vi "HFRR ADV v039 new software.vi"() -> ()   [LabVIEW 2025] (continued)
                n2173 = Number To Fractional String(number=w2771, width (-)=i16 10 ("precision (6)"), precision (6)=i16 5) -> (F-format string=w2865:string)  [unwired: 1 in]
                n2174 = Number To Fractional String(number=w2771, width (-)=i16 10 ("precision (6)"), precision (6)=i16 5) -> (F-format string=w2866:string)  [unwired: 1 in]
                n2175 = Concatenate Strings("[CHH]" ("string"), w2792, "-Humidity Dry" ("string"), "\r") -> (w2786:string)
                n2176 = Concatenate Strings("[CHG]" ("string"), w2797, "-Humidity Wet" ("string"), "\r") -> (w2787:string)
                n2177 = Concatenate Strings("[CHD]" ("string"), w2808, "-Power +" ("string"), "\r") -> (w2790:string)
                n2178 = Concatenate Strings("[CHC]" ("string"), w2814, "-Language Selection" ("string"), "\r") -> (w2811:string)
                n2179 = Concatenate Strings("[CHA]" ("string"), w2825, "- Stroke Gain" ("string"), "\r") -> (w2819:string)
                n2180 = Concatenate Strings("[CHF]" ("string"), w2800, "-Heater" ("string"), "\r") -> (w2788:string)
                n2181 = Concatenate Strings("[CHE]" ("string"), w2805, "-Power_" ("string"), "\r") -> (w2789:string)
                n2182 = Concatenate Strings("[CH8]" ("string"), w2826, "- Displacement Gain" ("string"), "\r") -> (w2829:string)
                n2183 = Concatenate Strings("[CH7]" ("string"), w2833, "- file path" ("string"), "\r") -> (w2836:string)
                n2184 = Concatenate Strings("[CH6]" ("string"), w2773, "- Visa Due" ("string"), "\r") -> (w2837:string)
                n2185 = Concatenate Strings("[CH5]" ("string"), w2774, "- Visa Uno" ("string"), "\r") -> (w2842:string)
                n2186 = Concatenate Strings("[CH4]" ("string"), w2853, " - AIR TEMP" ("string"), "\r") -> (w2849:string)
                n2187 = Concatenate Strings("[CH3]" ("string"), w2859, " - Humidity" ("string"), "\r") -> (w2856:string)
                n2188 = Concatenate Strings("[CH2]" ("string"), w2865, " - TEMPERATURE" ("string"), "\r") -> (w2863:string)
                n2189 = Concatenate Strings("[CH1]" ("string"), w2866, " - FF" ("string"), "\r") -> (w2864:string)
                n2190 = Concatenate Strings(w2864, w2863, w2856, w2849, w2842, w2837, w2836, w2829, w2819, w2811, w2790, w2789, w2788, w2787, w2786) -> (w2775:string)
                "gain" <- w2775
              }
              frame #1 {
                w2877 = 0.0 ("number")
                n2191 = local read "Camera Port :"() -> (w2880:string)
                n2192 = local read "C3 :"() -> (w2888:refnum<visa-resource-name>)
                n2193 = local read "Com Port 3"() -> (w2889:refnum<visa-resource-name>)
                n2194 = Concatenate Strings("[CH8]" ("string"), w2880, "- Visa Camera" ("string"), "\r") -> (w2879:string)
                n2195 = Concatenate Strings("[CH7]" ("string"), w2888, "- Visa Humidity" ("string"), "\r") -> (w2884:string)
                n2196 = Number To Fractional String(number=w2877, width (-)=i16 10 ("precision (6)"), precision (6)=i16 5) -> (F-format string=w2904:string)  [unwired: 1 in]
                n2197 = Concatenate Strings("[CHL]" ("string"), w2889, "- Visa humid" ("string"), "\r") -> (w2892:string)
                n2198 = Number To Fractional String(number=w2877, width (-)=i16 10 ("precision (6)"), precision (6)=i16 5) -> (F-format string=w2911:string)  [unwired: 1 in]
                n2199 = Concatenate Strings("[SNO]" ("string"), "" ("string"), "-" ("string"), "\r") -> (w2897:string)
                n2200 = Concatenate Strings("[CHK]" ("string"), w2904, "-TEMP INTERCEPT" ("string"), "\r") -> (w2900:string)
                n2201 = Concatenate Strings("[CHJ]" ("string"), w2911, "-AIR TEMP INTERCEPT" ("string"), "\r") -> (w2901:string)
                n2202 = String To Path(string="C:\\LAB-IQ\\calibrate WO 2465.dcf") -> (path=w2890:path)
                n2203 = Concatenate Strings(w2916, w2901, w2900, w2897, w2892, w2884, w2879) -> (w2915:string)
                n2204 = call <vilib>:"Write Characters To File.vi"("append to file? (new file:F)"=FALSE, "character string"=w2915, "file path (dialog if empty)"=w2890) -> ()  [unwired: 2 in, 1 out]
              }
              frame #2 {
                n2205 = local write "Lan flag"(0.0 ("Lan flag")) -> ()
                n2206 = local write "conststatus"(0.0 ("rpm value : 2")) -> ()
                n2207 = local write "SAVE"(FALSE ("OK Button 14")) -> ()
              }
            }
          }
        }
        n2208 = property on="Language Selection" class="Enum (strict)"("Visible"=w2712) -> ()  [unwired: 2 in, 2 out]
        n2209 = property on="SPEED OUT:" class="DigNum (strict)"("Disabled"=w2713) -> ()  [unwired: 2 in, 2 out]
      }
    }
    n2210 = case shown="False" w2239 {
      frame False {
        n2211 = local read "stopT"() -> (w2927:bool)
        n2212 = case shown="True" w2927 {
          frame False {
          }
          frame True {
            n2213 = local write "stopT"(FALSE) -> ()
          }
        }
      }
      frame True {
        "stopT" <- TRUE
      }
    }
    n2214 = case shown="True" w2229 {
      frame False {
        n2215 = property on="Password 2" class="Str"("Visible"=FALSE) -> ()  [unwired: 2 in, 2 out]
        n2216 = local write "Password 2"("" ("Password")) -> ()
      }
      frame True {
        n2217 = property on="Password 2" class="Str"("Visible"=TRUE) -> ()  [unwired: 2 in, 2 out]
        n2218 = Equal?(x="Password 2", y="HFRR1234") -> (x = y?=w2252:bool)
        n2219 = case shown="True" w2252 {
          tunnel: "Password 2" -> [w2255 _]
          frame False {
            n2220 = String Length(string=w2255) -> (length=w2256:i32)
            n2221 = Greater Than 0?(x=w2256) -> (x > 0?=w2254:bool)
            n2222 = case shown="False" w2254 {
              frame False {
                n2223 = property on="Password 2" class="Str"("Caption.Text"="Password (Advance Setting)") -> ()  [unwired: 2 in, 2 out]
              }
              frame True {
                n2224 = property on="Password 2" class="Str"("Caption.Text"="Incorrect Password!") -> ()  [unwired: 2 in, 2 out]
              }
            }
          }
          frame True {
            n2225 = local write "EDIT 2"(FALSE ("EDIT 2")) -> ()
            n2226 = local write "Password 2"("" ("Password")) -> ()
            n2227 = local write "Main Tab"(T2."Advance" ("Main Tab")) -> ()
            n2228 = local write "Main Dashboard Buttons"(T1."Advance" ("Main Dashboard Buttons")) -> ()
          }
        }
      }
    }
    n2229 = case shown="\"Acquire\", Default" w2235 {
      frame "Acquire", Default {
        # "Elapsed time\ncof\nstroke\nAir temp\nTemp\nHumidity"
        n2230 = local read "RUN"() -> (w2934:bool)
        n2231 = stacked-sequence {
          frame #0 {
            n2232 = case shown="True" "RST FF" {
              frame False {
              }
              frame True {
                w3011 = 0.0 ("X Scale.Range:Maximum")
                n2233 = property on="Frictional Force ( N )" class="WFChart (strict)"("XScale.Maximum"=600.0 ("X Scale.Range:Maximum"), "XScale.Minimum"=w3011, "YScale.Maximum"=10.0 ("Y Scale.Range:Maximum"), "YScale.Minimum"=w3011) -> ()  [unwired: 2 in, 2 out]
              }
            }
          }
          frame #1 {
            n2234 = case shown="True" "RST TEMP" {
              frame False {
              }
              frame True {
                n2235 = property on="Temperature ( Deg C )" class="WFChart (strict)"("XScale.Minimum"=0.0 ("X Scale.Range:Minimum"), "XScale.Maximum"=600.0 ("X Scale.Range:Maximum"), "YScale.Minimum"=0.0 ("Y Scale.Range:Minimum"), "YScale.Maximum"=100.0 ("Y Scale.Range:Maximum")) -> ()  [unwired: 2 in, 2 out]
              }
            }
          }
          frame #2 {
            n2236 = case shown="True" "RSTCOF" {
              frame False {
              }
              frame True {
                n2237 = property on="Coefficient of Friction" class="WFChart (strict)"("XScale.Minimum"=0.0 ("X Scale.Range:Minimum"), "XScale.Maximum"=600.0 ("X Scale.Range:Maximum"), "YScale.Maximum"=1.0 ("X Scale.Range:Minimum"), "YScale.Minimum"=0.0 ("X Scale.Range:Minimum")) -> ()  [unwired: 2 in, 2 out]
              }
            }
          }
          frame #3 {
            n2238 = case shown="True" "RSTCOF 2" {
              frame False {
              }
              frame True {
                (unwired) 100.0 ("Y Scale.Range:Maximum")
                (unwired) 0.0 ("Y Scale.Range:Minimum")
                (unwired) 600.0 ("X Scale.Range:Maximum")
                (unwired) 0.0 ("X Scale.Range:Minimum")
              }
            }
          }
          frame #4 {
            n2239 = case shown="True" "RSTCOF 3" {
              frame False {
              }
              frame True {
                n2240 = property on="Electrical Contact Resistance ( % )" class="WFChart (strict)"("XScale.Minimum"=0.0 ("X Scale.Range:Minimum"), "XScale.Maximum"=600.0 ("X Scale.Range:Maximum"), "YScale.Minimum"=0.0 ("Y Scale.Range:Minimum"), "YScale.Maximum"=100.0 ("Y Scale.Range:Maximum")) -> ()  [unwired: 2 in, 2 out]
              }
            }
          }
        }
        n2241 = case shown="False" w2934 {
          frame False {
          }
          frame True {
          }
        }
        n2242 = disable-structure shown="Disabled" {
          frame Disabled {
            n2243 = local read "RUN"() -> (w2941:bool)
            n2244 = local read "Flag"() -> (w2944:dbl)
            n2245 = Not(x=w2941) -> (.not. x?=w2940:bool)
            n2246 = Equal?(x=w2944, y=10.0) -> (x = y?=w2942:bool)
            n2247 = And(x=w2942, y=w2940) -> (x .and. y?=w2939:bool)
            n2248 = case shown="True" w2939 {
              frame False {
              }
              frame True {
                w2945 = FALSE ("Heater Button")
                n2249 = local write "Humidity"(w2945) -> ()
                n2250 = local write "Heater Button"(w2945) -> ()
              }
            }
          }
          frame Enabled {
          }
        }
        n2251 = local read "RUN"() -> (w2938:bool)
        n2252 = case shown="False" w2938 {
          tunnel: [FALSE ("TEST RUNNING") TRUE ("TEST RUNNING")] -> w2937
          frame False {
            w3030 = 0.0 ("Flag")
            n2253 = local write "Elapsed time"(0.0 ("elapsedtime")) -> ()
            n2254 = local write "Time Remaining"(w3030) -> ()
            n2255 = local write "Flag"(w3030) -> ()
            n2256 = local write "Remaining Time"(w3030) -> ()
          }
          frame True {
            n2257 = local write "Flag"(10.0 ("Flag")) -> ()
          }
        }
        n2258 = local read "AIR TEMP"() -> (w2932:dbl)
        n2259 = Greater Or Equal?(x=w2932, y=15.0) -> (x >= y?=w2933:bool)
        "powstat" <- w2933
        n2260 = case shown="True" "Save & Continue" {
          frame False {
          }
          frame True {
            n2261 = local read "USER ID"() -> (w3339:string)
            n2262 = local read "FILE"() -> (w3347:string)
            n2263 = String Length(string=w3339) -> (length=w3342:i32)
            n2264 = String Length(string=w3347) -> (length=w3345:i32)
            n2265 = Greater?(x=w3342, y=0) -> (0:w3341:bool)
            n2266 = Greater?(x=w3345, y=0) -> (0:w3344:bool)
            n2267 = And(x=w3344, y=w3341) -> (x .and. y?=w3340:bool)
            n2268 = case shown="True" w3340 {
              frame False {
                n2269 = stacked-sequence {
                  frame #0 {
                    n2270 = One Button Dialog(message="Please Enter a File Name and Operator ID to save data !", button name ("OK")="Ok") -> ()  [unwired: 1 out]
                  }
                  frame #1 {
                    n2271 = local write "Save & Continue"(FALSE ("OK Button")) -> ()
                  }
                }
                n2272 = local write "Save & Continue"(FALSE ("OK Button")) -> ()
              }
              frame True {
                n2273 = stacked-sequence {
                  frame #0 {
                    n2274 = local read "FILE"() -> (w3353:string)
                    n2275 = call "file check.vi"("file name in"=w3353) -> ("file name out"=w3352:string)  [unwired: 9 in, 1 out]
                    n2276 = call <vilib>:"Application Directory.vi"() -> ("Application Directory"=w3363:path)
                    n2277 = Build Path(base path=w3363, name or relative path="data") -> (appended path=w3362:path)
                    n2278 = call <vilib>:"Trim Whitespace.vi"("string"=w3352) -> ("trimmed string"=w3360:string)  [unwired: 1 in]
                    n2279 = call <vilib>:"Trim Whitespace.vi"("string"=w3352) -> ("trimmed string"=w3361:string)  [unwired: 1 in]
                    n2280 = List Folder(path=w3362) -> (folder names=w3358:string[])  [unwired: 3 in, 3 out]
                    n2281 = Match Pattern(string=w3360, regular expression="_(") -> (before substring=w3357:string)  [unwired: 1 in, 3 out]
                    n2282 = Equal?(x=w3358, y=w3357) -> (x = y?=w3366:bool[])
                    n2283 = for {
                      tunnel: w3358 -> [w3372] mode=indexing
                      tunnel: w3357 -> [w3370]
                      shift-right: [w3368] -> w3355
                      shift-left: bool[] [] -> [w3369]
                      n2284 = Match Pattern(string=w3372, regular expression="_(") -> (before substring=w3371:string)  [unwired: 1 in, 3 out]
                      n2285 = Equal?(x=w3371, y=w3370) -> (x = y?=w3367:bool)
                      n2286 = case shown="True" w3367 {
                        tunnel: w3367 -> [_ w3375]
                        tunnel: w3369 -> [w3374 w3377]
                        tunnel: [w3374 w3376] -> w3368
                        frame False {
                        }
                        frame True {
                          n2287 = Insert Into Array(array=w3377, new element=w3375) -> (w3376:bool[])  [unwired: 1 in]
                        }
                      }
                    }
                    n2288 = Or Array Elements(Boolean array=w3366) -> (logical OR=w3365:bool)
                    n2289 = Array Size(array=w3355) -> (size(s)=w3354:i32)
                    n2290 = case shown="True" w3365 {
                      tunnel: w3361 -> [_ w3385]
                      tunnel: w3354 -> [_ w3378]
                      frame False {
                      }
                      frame True {
                        n2291 = Number To Decimal String(number=w3378) -> (decimal integer string=w3381:string)  [unwired: 1 in]
                        n2292 = Search/Split String(string=w3385, search string/char (-)="_(" ("regular expression")) -> (substring before match=w3383:string)  [unwired: 1 in, 2 out]
                        n2293 = Concatenate Strings(w3383, "_(" ("regular expression"), w3381, ")" ("regular expression")) -> (w3379:string)
                        n2294 = local write "FILE"(w3379) -> ()
                      }
                    }
                  }
                  frame #1 {
                    w3388 = 0.0
                    w3401 = cluster{"y":dbl, dbl, "y":dbl}[] [] ("History Data")
                    w3402 = FALSE ("Heater Button")
                    (unwired) ")!" ("string")
                    (unwired) ")" ("string")
                    w3400 = dbl[] [] ("History Data")
                    w3406 = "\r"
                    # "C:\\WinDucom\\Data\\"
                    # "C:\\LAB-IQ-NXT\\data"
                    n2295 = local write "Humidity ( %RH )"(w3388) -> ()
                    n2296 = local write "Frequency ( Hz )"(w3388) -> ()
                    n2297 = local write "Stroke 3"(w3388) -> ()
                    n2298 = local write "Set Temp 2"(65.0 ("Set Temp 2")) -> ()
                    n2299 = local write "speedop"(0.0 ("PIDclk 2")) -> ()
                    n2300 = local write "AIR TEMP"(w3388) -> ()
                    n2301 = local write "Stroke 4"(w3388) -> ()
                    n2302 = local write "clk"(0.0 ("clk")) -> ()
                    n2303 = local write "COF 2"(w3388) -> ()
                    n2304 = local write "TEMP"(w3388) -> ()
                    n2305 = local write "ecr 3"(w3388) -> ()
                    n2306 = local write "FF 2"(w3388) -> ()
                    n2307 = local write "FF 3"(w3388) -> ()
                    n2308 = property on="Temperature ( Deg C )" class="WFChart (strict)"("History Data"=w3400) -> ()  [unwired: 2 in, 2 out]
                    n2309 = property on="Electrical Contact Resistance ( % )" class="WFChart (strict)"("History Data"=w3400) -> ()  [unwired: 2 in, 2 out]
                    n2310 = property on="Frictional Force ( N )" class="WFChart (strict)"("History Data"=w3400) -> ()  [unwired: 2 in, 2 out]
                    n2311 = property on="Coefficient of Friction" class="WFChart (strict)"("History Data"=w3400) -> ()  [unwired: 2 in, 2 out]
                    n2312 = property on="Humidity ( %RH ) 2" class="WFChart (strict)"("History Data"=w3400) -> ()  [unwired: 2 in, 2 out]
                    n2313 = property on="Temperature ( Deg C )" class="WFChart (strict)"("History Data"=w3400) -> ()  [unwired: 2 in, 2 out]
                    n2314 = property on="Electrical Contact Resistance ( % )" class="WFChart (strict)"("History Data"=w3400) -> ()  [unwired: 2 in, 2 out]
                    n2315 = property on="Frictional Force ( N )" class="WFChart (strict)"("History Data"=w3400) -> ()  [unwired: 2 in, 2 out]
                    n2316 = property on="Coefficient of Friction" class="WFChart (strict)"("History Data"=w3400) -> ()  [unwired: 2 in, 2 out]
                    n2317 = property on="Electrical Contact Resistance ( % )" class="WFChart (strict)"("History Data"=w3400) -> ()  [unwired: 2 in, 2 out]
                    n2318 = property on="Frictional Force ( N )" class="WFChart (strict)"("History Data"=w3400) -> ()  [unwired: 2 in, 2 out]
                    n2319 = property on="Coefficient of Friction" class="WFChart (strict)"("History Data"=w3400) -> ()  [unwired: 2 in, 2 out]
                    n2320 = property on="Stroke ( mm )" class="WFChart (strict)"("History Data"=w3401) -> ()  [unwired: 2 in, 2 out]
                    n2321 = property on="Stroke ( mm )" class="WFChart (strict)"("History Data"=w3401) -> ()  [unwired: 2 in, 2 out]
                    n2322 = local write "Humidity"(w3402) -> ()
                    n2323 = local write "Heater Button"(w3402) -> ()
                    n2324 = local read "FILE"() -> (w3396:string)
                    n2325 = disable-structure shown="Enabled" {
                      disable-tunnel: [w3440 _] -> w3387
                      frame Enabled {
                        n2326 = local read "NORMAL LOAD"() -> (w3440:dbl)
                      }
                      frame Disabled {
                      }
                    }
                    n2327 = call "file check.vi"("file name in"=w3396) -> ("error out"=w3399:errorcluster, "file name out"=w3393:string)  [unwired: 9 in]
                    n2328 = call "FILE PATH CREATION.vi"("error in"=w3399, "FILE NAME :"=w3393) -> ("FILE OUT"=w3392:path)  [unwired: 8 in, 1 out]
                    n2329 = Concatenate Strings(w3393, ".dgf" ("Substring")) -> (w3398:string)
                    n2330 = Concatenate Strings(w3393, ".duf" ("Substring")) -> (w3394:string)
                    n2331 = Multiply(x=w3387, y=1.0) -> (x*y=w3419:dbl)
                    n2332 = Build Path(base path=w3392, name or relative path=w3398) -> (appended path=w3391:path)
                    n2333 = Build Path(base path=w3392, name or relative path=w3394) -> (appended path=w3390:path)
                    n2334 = Number To Fractional String(number=w3419, width (-)=i16 5, precision (6)=i16 2) -> (F-format string=w3427:string)  [unwired: 1 in]
                    n2335 = local read "tested by"() -> (w3386:string)
                    n2336 = local read "Fuel Discription :"() -> (w3415:string)
                    n2337 = local read "Batch Ref Num :"() -> (w3404:string)
                    n2338 = Get Date/Time String(date format (0)=enum16{"short", "long", "abbreviated"}."short") -> (date string=w3438:string, time string=w3435:string)  [unwired: 2 in]
                    n2339 = local read "Remarks :"() -> (w3414:string)
                    n2340 = Concatenate Strings("Load :- " ("Substring"), w3427, " grams ," ("Substring")) -> (w3426:string)
                    n2341 = local read "String 41"() -> (w3407:string)
                    n2342 = Concatenate Strings(w3404) -> (w3403:string)
                    n2343 = Concatenate Strings(w3386) -> (w3410:string)
                    n2344 = Concatenate Strings(w3415) -> (w3416:string)
                    n2345 = Concatenate Strings("(" ("Substring"), w3438, ")" ("Substring"), w3435) -> (w3409:string)
                    "concatenated string" <- w3409
                    n2346 = Concatenate Strings(w3414, "," ("string")) -> (w3413:string)
                    n2347 = Concatenate Strings("  TIME;      COF;       STROKE;     AIR TEMP;  TEMP;  HUMIDITY;  ECR; PID-OUT; FREQUENCY" ("Substring"), "\r") -> (w3422:string)
                    n2348 = Concatenate Strings(w3407, w3406, "Fuel Discription :-" ("Substring"), w3416, w3406, w3426, w3406, "Batch Ref Num :-" ("Substring"), w3403, w3406, " Remarks :- " ("Substring"), w3413, w3406, " Date :- " ("Substring"), w3409, w3406, "Tested By :-" ("Substring"), w3410) -> (w3420:string)
                    "REMARKS" <- w3420
                    n2349 = call <vilib>:"Write Characters To File.vi"("append to file? (new file:F)"=FALSE, "character string"=w3420, "file path (dialog if empty)"=w3390) -> ()  [unwired: 2 in, 1 out]
                    n2350 = call <vilib>:"Write Characters To File.vi"("append to file? (new file:F)"=FALSE, "character string"=w3422, "file path (dialog if empty)"=w3391) -> ()  [unwired: 2 in, 1 out]
                  }
                  frame #2 {
                    n2351 = local write "Cycles elapsed"(0 ("Cycles elapsed")) -> ()
                    n2352 = local write "cyclecount"(0 ("cyclecount")) -> ()
                    n2353 = local write "autostrtflg"(TRUE ("autostrtflg")) -> ()
                    n2354 = local write "Save"(FALSE ("Save")) -> ()
                    n2355 = local write "Save & Continue"(FALSE ("OK")) -> ()
                    n2356 = Get Date/Time In Seconds() -> (seconds since 1Jan1904=w3445:timestamp)
                    n2357 = To Double Precision Float(number=w3445) -> (double precision float=w3444:dbl)
                    n2358 = local write "acq timer"(w3444) -> ()
                    n2359 = One Button Dialog(message="Please ensure sample is mounted properly and machine is ready in all aspects for testing !", button name ("OK")="Ok") -> ()  [unwired: 1 out]
                  }
                  frame #3 {
                    n2360 = stacked-sequence {
                      frame #0 {
                        n2361 = local write "Main Dashboard Buttons"(T1."Dashboard" ("Main Dashboard Buttons")) -> ()
                        n2362 = local write "Main Tab"(T2."Acquire" ("Main Tab")) -> ()
                      }
                      frame #1 {
                        n2363 = local write "EVENT LOG"("" ("EVENT LOG")) -> ()
                      }
                      frame #2 {
                        n2364 = Wait (ms)(milliseconds to wait=u32 50) -> ()  [unwired: 1 out]
                      }
                      frame #3 {
                        n2365 = disable-structure shown="Disabled" {
                          frame Disabled {
                            n2366 = local read "EVENT LOG"() -> (w3457:string)
                            n2367 = call "Event Log.vi"("Content"="Test Details", "EVENT LOG"=w3457) -> ("EVENT LOG"=w3456:string)  [unwired: 8 in, 1 out]
                            n2368 = local write "EVENT LOG"(w3456) -> ()
                          }
                          frame Enabled {
                          }
                        }
                      }
                      frame #4 {
                        n2369 = Wait (ms)(milliseconds to wait=u32 50) -> ()  [unwired: 1 out]
                      }
                      frame #5 {
                        n2370 = local read "FILE"() -> (w3459:string)
                        n2371 = Concatenate Strings("File Name :" ("Content"), w3459) -> (w3460:string)
                        n2372 = local read "EVENT LOG"() -> (w3463:string)
                        n2373 = call "Event Log.vi"("Content"=w3460, "EVENT LOG"=w3463) -> ("EVENT LOG"=w3462:string)  [unwired: 8 in, 1 out]
                        n2374 = local write "EVENT LOG"(w3462) -> ()
                      }
                      frame #6 {
                        n2375 = Wait (ms)(milliseconds to wait=u32 50) -> ()  [unwired: 1 out]
                      }
                      frame #7 {
                        n2376 = local read "Batch Ref Num :"() -> (w3465:string)
                        n2377 = Concatenate Strings("Batch Ref No :" ("Content"), w3465) -> (w3466:string)
                        n2378 = local read "EVENT LOG"() -> (w3469:string)
                        n2379 = call "Event Log.vi"("Content"=w3466, "EVENT LOG"=w3469) -> ("EVENT LOG"=w3468:string)  [unwired: 8 in, 1 out]
                        n2380 = local write "EVENT LOG"(w3468) -> ()
                      }
                      frame #8 {
                        n2381 = Wait (ms)(milliseconds to wait=u32 50) -> ()  [unwired: 1 out]
                      }
                      frame #9 {
                        n2382 = local read "tested by"() -> (w3471:string)
                        n2383 = Concatenate Strings("Tested By :" ("Content"), w3471) -> (w3472:string)
                        n2384 = local read "EVENT LOG"() -> (w3475:string)
                        n2385 = call "Event Log.vi"("Content"=w3472, "EVENT LOG"=w3475) -> ("EVENT LOG"=w3474:string)  [unwired: 8 in, 1 out]
                        n2386 = local write "EVENT LOG"(w3474) -> ()
                      }
                      frame #10 {
                        n2387 = Wait (ms)(milliseconds to wait=u32 50) -> ()  [unwired: 1 out]
                      }
                      frame #11 {
                        n2388 = local read "TEST STANDARD"() -> (w3478:T3)
                        n2389 = case shown="\"ASTM D6079\", Default" w3478 {
                          tunnel: ["ASTM D6079" "ISO 12156" "CEC F-096-A-06" "Custom"] -> w3477
                          frame "ASTM D6079", Default {
                          }
                          frame "ISO 12156" {
                          }
                          frame "CEC F-096-A-06" {
                          }
                          frame "Custom" {
                          }
                        }
                        n2390 = Concatenate Strings("Test Standard :" ("Content"), w3477) -> (w3479:string)
                        n2391 = local read "EVENT LOG"() -> (w3482:string)
                        n2392 = call "Event Log.vi"("Content"=w3479, "EVENT LOG"=w3482) -> ("EVENT LOG"=w3481:string)  [unwired: 8 in, 1 out]
                        n2393 = local write "EVENT LOG"(w3481) -> ()
                      }
                      frame #12 {
                        n2394 = Wait (ms)(milliseconds to wait=u32 50) -> ()  [unwired: 1 out]
                      }
                      frame #13 {
                        n2395 = local read "Fuel Discription :"() -> (w3488:string)
                        n2396 = Concatenate Strings("Fuel Description :" ("Content"), w3488) -> (w3489:string)
                        n2397 = local read "EVENT LOG"() -> (w3492:string)
                        n2398 = call "Event Log.vi"("Content"=w3489, "EVENT LOG"=w3492) -> ("EVENT LOG"=w3491:string)  [unwired: 8 in, 1 out]
                        n2399 = local write "EVENT LOG"(w3491) -> ()
                      }
                      frame #14 {
                        n2400 = Wait (ms)(milliseconds to wait=u32 50) -> ()  [unwired: 1 out]
                      }
                      frame #15 {
                        n2401 = local read "Remarks :"() -> (w3494:string)
                        n2402 = Concatenate Strings("Remarks :" ("Content"), w3494) -> (w3495:string)
                        n2403 = local read "EVENT LOG"() -> (w3498:string)
                        n2404 = call "Event Log.vi"("Content"=w3495, "EVENT LOG"=w3498) -> ("EVENT LOG"=w3497:string)  [unwired: 8 in, 1 out]
                        n2405 = local write "EVENT LOG"(w3497) -> ()
                      }
                      frame #16 {
                        n2406 = Wait (ms)(milliseconds to wait=u32 50) -> ()  [unwired: 1 out]
                      }
                      frame #17 {
                        n2407 = local read "USER ID"() -> (w3500:string)
                        n2408 = Concatenate Strings("Operator ID :" ("Content"), w3500) -> (w3502:string)
                        n2409 = local read "EVENT LOG"() -> (w3504:string)
                        n2410 = call "Event Log.vi"("Content"=w3502, "EVENT LOG"=w3504) -> ("EVENT LOG"=w3503:string)  [unwired: 8 in, 1 out]
                        n2411 = local write "EVENT LOG"(w3503) -> ()
                      }
                      frame #18 {
                        n2412 = Wait (ms)(milliseconds to wait=u32 50) -> ()  [unwired: 1 out]
                      }
                      frame #19 {
                        n2413 = disable-structure shown="Disabled" {
                          frame Disabled {
                            n2414 = local read "EVENT LOG"() -> (w3508:string)
                            n2415 = call "Event Log.vi"("Content"="Test Parameter", "EVENT LOG"=w3508) -> ("EVENT LOG"=w3507:string)  [unwired: 8 in, 1 out]
                            n2416 = local write "EVENT LOG"(w3507) -> ()
                          }
                          frame Enabled {
                          }
                        }
                      }
                      frame #20 {
                        n2417 = Wait (ms)(milliseconds to wait=u32 50) -> ()  [unwired: 1 out]
                      }
                      frame #21 {
                        n2418 = local read "Set Hz"() -> (w3512:dbl)
                        n2419 = Number To Fractional String(number=w3512, precision (6)=i16 2) -> (F-format string=w3511:string)  [unwired: 2 in]
                        n2420 = Concatenate Strings("Set Frequency [Hz] :" ("Content"), w3511) -> (w3514:string)
                        n2421 = local read "EVENT LOG"() -> (w3516:string)
                        n2422 = call "Event Log.vi"("Content"=w3514, "EVENT LOG"=w3516) -> ("EVENT LOG"=w3515:string)  [unwired: 8 in, 1 out]
                        n2423 = local write "EVENT LOG"(w3515) -> ()
                      }
                      frame #22 {
                        n2424 = Wait (ms)(milliseconds to wait=u32 50) -> ()  [unwired: 1 out]
                      }
                      frame #23 {
                        n2425 = local read "NORMAL LOAD"() -> (w3519:dbl)
                        n2426 = Number To Fractional String(number=w3519, precision (6)=i16 2) -> (F-format string=w3520:string)  [unwired: 2 in]
                        n2427 = Concatenate Strings("Applied Load [grams] :" ("Content"), w3520) -> (w3522:string)
                        n2428 = local read "EVENT LOG"() -> (w3524:string)
                        n2429 = call "Event Log.vi"("Content"=w3522, "EVENT LOG"=w3524) -> ("EVENT LOG"=w3523:string)  [unwired: 8 in, 1 out]
                        n2430 = local write "EVENT LOG"(w3523) -> ()
                      }
                      frame #24 {
                        n2431 = Wait (ms)(milliseconds to wait=u32 50) -> ()  [unwired: 1 out]
                      }
                      frame #25 {
                        n2432 = local read "Set Strk"() -> (w3527:dbl)
                        n2433 = Number To Fractional String(number=w3527, precision (6)=i16 2) -> (F-format string=w3528:string)  [unwired: 2 in]
                        n2434 = Concatenate Strings("Set Stroke [mm] :" ("Content"), w3528) -> (w3530:string)
                        n2435 = local read "EVENT LOG"() -> (w3532:string)
                        n2436 = call "Event Log.vi"("Content"=w3530, "EVENT LOG"=w3532) -> ("EVENT LOG"=w3531:string)  [unwired: 8 in, 1 out]
                        n2437 = local write "EVENT LOG"(w3531) -> ()
                      }
                      frame #26 {
                        n2438 = Wait (ms)(milliseconds to wait=u32 50) -> ()  [unwired: 1 out]
                      }
                      frame #27 {
                        n2439 = local read "Set Temp"() -> (w3535:dbl)
                        n2440 = Number To Fractional String(number=w3535, precision (6)=i16 2) -> (F-format string=w3536:string)  [unwired: 2 in]
                        n2441 = Concatenate Strings("Set Temperature [deg C] :" ("Content"), w3536) -> (w3538:string)
                        n2442 = local read "EVENT LOG"() -> (w3540:string)
                        n2443 = call "Event Log.vi"("Content"=w3538, "EVENT LOG"=w3540) -> ("EVENT LOG"=w3539:string)  [unwired: 8 in, 1 out]
                        n2444 = local write "EVENT LOG"(w3539) -> ()
                      }
                      frame #28 {
                        n2445 = Wait (ms)(milliseconds to wait=u32 50) -> ()  [unwired: 1 out]
                      }
                      frame #29 {
                        n2446 = local read "Set Rh"() -> (w3543:dbl)
                        n2447 = Number To Fractional String(number=w3543, precision (6)=i16 2) -> (F-format string=w3544:string)  [unwired: 2 in]
                        n2448 = Concatenate Strings("Set Humidity [%RH] :" ("Content"), w3544) -> (w3546:string)
                        n2449 = local read "EVENT LOG"() -> (w3548:string)
                        n2450 = call "Event Log.vi"("Content"=w3546, "EVENT LOG"=w3548) -> ("EVENT LOG"=w3547:string)  [unwired: 8 in, 1 out]
                        n2451 = local write "EVENT LOG"(w3547) -> ()
                      }
                      frame #30 {
                        n2452 = Wait (ms)(milliseconds to wait=u32 50) -> ()  [unwired: 1 out]
                      }
                      frame #31 {
                        n2453 = local read "test time"() -> (w3551:dbl)
                        n2454 = Number To Fractional String(number=w3551, precision (6)=i16 1) -> (F-format string=w3552:string)  [unwired: 2 in]
                        n2455 = Concatenate Strings("Test Duration [mins] :" ("Content"), w3552) -> (w3554:string)
                        n2456 = local read "EVENT LOG"() -> (w3556:string)
                        n2457 = call "Event Log.vi"("Content"=w3554, "EVENT LOG"=w3556) -> ("EVENT LOG"=w3555:string)  [unwired: 8 in, 1 out]
                        n2458 = local write "EVENT LOG"(w3555) -> ()
                      }
                      frame #32 {
                        w3557 = dbl[] [] ("History Data")
                        w3558 = cluster{"y":dbl, dbl, "y":dbl}[] [] ("History Data")
                        w3559 = FALSE ("Visible")
                        n2459 = property on="Stroke ( mm )" class="WFChart (strict)"("History Data"=w3558) -> ()  [unwired: 2 in, 2 out]
                        n2460 = property on="Humidity ( %RH ) 2" class="WFChart (strict)"("History Data"=w3557) -> ()  [unwired: 2 in, 2 out]
                        n2461 = property on="Temperature ( Deg C )" class="WFChart (strict)"("History Data"=w3557) -> ()  [unwired: 2 in, 2 out]
                        n2462 = property on="Electrical Contact Resistance ( % )" class="WFChart (strict)"("History Data"=w3557) -> ()  [unwired: 2 in, 2 out]
                        n2463 = property on="Frictional Force ( N )" class="WFChart (strict)"("History Data"=w3557) -> ()  [unwired: 2 in, 2 out]
                        n2464 = property on="Coefficient of Friction" class="WFChart (strict)"("History Data"=w3557) -> ()  [unwired: 2 in, 2 out]
                        n2465 = property on="Coefficient of Friction" class="WFChart (strict)"("History Data"=w3557) -> ()  [unwired: 2 in, 2 out]
                        n2466 = property on="Electrical Contact Resistance ( % )" class="WFChart (strict)"("History Data"=w3557) -> ()  [unwired: 2 in, 2 out]
                        n2467 = property on="Frictional Force ( N )" class="WFChart (strict)"("History Data"=w3557) -> ()  [unwired: 2 in, 2 out]
                        n2468 = property on="Stroke ( mm )" class="WFChart (strict)"("History Data"=w3558) -> ()  [unwired: 2 in, 2 out]
                        n2469 = property on="Temperature ( Deg C )" class="WFChart (strict)"("History Data"=w3557) -> ()  [unwired: 2 in, 2 out]
                        n2470 = property on="Service Password Log" class="Str"("Visible"=w3559) -> ()  [unwired: 2 in, 2 out]
                        n2471 = property on="Password 3" class="Clust (strict)"("Visible"=w3559) -> ()  [unwired: 2 in, 2 out]
                      }
                    }
                    "TEST FILE NAM,E SAVED" <- TRUE ("TEST FILE NAM,E SAVED")
                  }
                }
              }
            }
          }
        }
        n2472 = local write "Test \nStatus"(w2937) -> ()
        n2473 = local write "Save"(w2937) -> ()
        n2474 = local read "Main Tab"() -> (w2931:T2)
        n2475 = disable-structure shown="Disabled" {
          frame Disabled {
            n2476 = case shown="True" {
              selector: _ -> [_ _]
              frame False {
              }
              frame True {
                w2994 = TRUE ("Heater")
                n2477 = local write "Heater Button"(w2994) -> ()
                n2478 = local write "Humidity"(w2994) -> ()
                n2479 = local read "TEST STANDARD"() -> (w2992:T3)
                n2480 = local read "TEST STANDARD"() -> (w2997:T3)
                n2481 = Equal?(x=w2992, y=enum16{"ASTM D6079", "ISO 12156", "Custom"}."ASTM D6079" ("Test Standard")) -> (x = y?=w2991:bool)
                n2482 = Equal?(x=w2997, y=enum16{"ASTM D6079", "ISO 12156", "Custom"}."ISO 12156" ("Test Standard")) -> (x = y?=w2995:bool)
                n2483 = case shown="True" w2991 {
                  frame False {
                  }
                  frame True {
                    n2484 = local write "airtempflg"(TRUE ("airtempflg")) -> ()
                    n2485 = local write item#-1(FALSE ("Heater")) -> ()
                  }
                }
                n2486 = case shown="True" w2995 {
                  frame False {
                  }
                  frame True {
                    n2487 = local write "airtempflg"(FALSE ("airtempflg")) -> ()
                    n2488 = local write item#-1(TRUE ("Heater")) -> ()
                  }
                }
              }
            }
          }
          frame Enabled {
          }
        }
        n2489 = case shown="\"Acquire\"" w2931 {
          tunnel: w2933 -> [_ w3037]
          frame Default {
            w3036 = 0.0 ("output")
            n2490 = local write "Frequency ( Hz )"(w3036) -> ()
            n2491 = local write "PID-out"(w3036) -> ()
            n2492 = local write "STROKE Initialize"(TRUE ("STROKE Initialize")) -> ()
          }
          frame "Acquire" {
            n2493 = stacked-sequence {
              frame #0 {
                n2494 = local read "Auto Start Test"() -> (w3039:bool)
                n2495 = case shown="True" w3039 {
                  tunnel: "RUN" -> [w3060 w3063]
                  tunnel: [w3060 w3062] -> w3040
                  frame False {
                  }
                  frame True {
                    n2496 = local read "Auto Start Temp"() -> (w3061:bool)
                    n2497 = Or(x=w3063, y=w3061) -> (x .or. y?=w3062:bool)
                  }
                }
                n2498 = local read "clk"() -> (w3059:dbl)
                n2499 = local read "Save"() -> (w3055:bool)
                n2500 = Equal?(x=w3059, y=0.0) -> (x = y?=w3056:bool)
                n2501 = And(x=w3056, y=w3055) -> (x .and. y?=w3057:bool)
                n2502 = Not(x="Engage") -> (.not. x?=w3046:bool)
                n2503 = case shown="False" w3040 {
                  tunnel: [0.0 w3086] -> w3042
                  frame False {
                    (unwired) TRUE ("Visible")
                    n2504 = local read "Auto Start Test"() -> (w3067:bool)
                    n2505 = local write "Start Time"(TRUE ("Start Time")) -> ()
                    n2506 = property on="Stroke 2" class="DigNum (strict)"("Visible"=FALSE) -> ()  [unwired: 2 in, 2 out]
                    n2507 = case shown="False" w3067 {
                      frame False {
                        n2508 = property on="Heater Button" class="Bool (strict)"("DisabledEnum"=T19."Enabled" ("Disabled")) -> ()  [unwired: 2 in, 2 out]
                        n2509 = property on="Humidity" class="Bool (strict)"("DisabledEnum"=T19."Enabled" ("Disabled")) -> ()  [unwired: 2 in, 2 out]
                      }
                      frame True {
                      }
                    }
                    n2510 = case shown="False" "TestCompFlg" {
                      frame False {
                        n2511 = local read "StartFlg"() -> (w3075:bool)
                        n2512 = case shown="True" w3075 {
                          frame False {
                          }
                          frame True {
                            n2513 = stacked-sequence {
                              frame #0 {
                                n2514 = local read "EVENT LOG"() -> (w3079:string)
                                n2515 = call "Event Log.vi"("Content"="Test was interrupted", "EVENT LOG"=w3079) -> ("EVENT LOG"=w3080:string)  [unwired: 8 in, 1 out]
                                n2516 = local write "EVENT LOG"(w3080) -> ()
                                n2517 = property on="RUN" class="Bool (strict)"("Visible"=TRUE) -> ()  [unwired: 2 in, 2 out]
                                n2518 = property on="Auto Start Test" class="Bool (strict)"("Visible"=TRUE) -> ()  [unwired: 2 in, 2 out]
                              }
                              frame #1 {
                                w3082 = FALSE ("StartFlg")
                                n2519 = property on="Heater Button" class="Bool (strict)"("Val(Sgnl)"=FALSE ("Value (Signaling)")) -> ()  [unwired: 2 in, 2 out]
                                n2520 = local write "Heater Button"(w3082) -> ()
                                n2521 = local write "StartFlg"(w3082) -> ()
                                n2522 = local write "Humidity"(w3082) -> ()
                              }
                              frame #2 {
                                n2523 = local write "Due Write"("VC;0" ("Command")) -> ()
                              }
                              frame #3 {
                                n2524 = Wait (ms)(milliseconds to wait=u32 1500) -> ()  [unwired: 1 out]
                              }
                              frame #4 {
                                n2525 = local write "Due Write"("HE;0" ("Command")) -> ()
                              }
                            }
                          }
                        }
                      }
                      frame True {
                      }
                    }
                    n2526 = local write "String 14"("Test will autostart once parameters reach the set value." ("String 14")) -> ()
                  }
                  frame True {
                    (unwired) FALSE ("Visible")
                    n2527 = property on="Stroke 2" class="DigNum (strict)"("Visible"=TRUE) -> ()  [unwired: 2 in, 2 out]
                    n2528 = property on="STOP 2" class="Bool (strict)"("Disabled"=u8 2) -> ()  [unwired: 2 in, 2 out]
                    n2529 = local write "String 14"(" Running....." ("String 14")) -> ()
                    n2530 = property on="Heater Button" class="Bool (strict)"("DisabledEnum"=T19."Disabled and Grayed Out" ("Disabled")) -> ()  [unwired: 2 in, 2 out]
                    n2531 = property on="Humidity" class="Bool (strict)"("DisabledEnum"=T19."Disabled and Grayed Out" ("Disabled")) -> ()  [unwired: 2 in, 2 out]
                    n2532 = case shown="True" "Start Time" {
                      selector: "Start Time" -> [_ w3105]
                      frame False {
                      }
                      frame True {
                        n2533 = Not(x=w3105) -> (.not. x?=w3104:bool)
                        n2534 = local write "Start Time"(w3104) -> ()
                        n2535 = local read "EVENT LOG"() -> (w3106:string)
                        n2536 = call "Event Log.vi"("Content"="Test in progress", "EVENT LOG"=w3106) -> ("EVENT LOG"=w3108:string)  [unwired: 8 in, 1 out]
                        n2537 = local write "EVENT LOG"(w3108) -> ()
                      }
                    }
                    n2538 = disable-structure shown="Enabled" {
                      disable-tunnel: [w3097 w3103] -> w3086
                      frame Disabled {
                        n2539 = local read "Set Hz"() -> (w3100:dbl)
                        n2540 = call <vilib>:"Uniform White Noise Waveform.vi"() -> ("signal out"=w3099:waveform(dbl))  [unwired: 10 in, 1 out]
                        n2541 = Random Number (0-1)() -> (number: 0 to 1=w3096:dbl)
                        n2542 = Add(x=w3100, y=w3099) -> (x+y=w3098:waveform(dbl))
                        n2543 = Multiply(x=ext 0.01 ("y"), y=w3096) -> (x*y=w3094:ext)
                        n2544 = Multiply(x=w3098, y=w3094) -> (x*y=w3097:waveform(ext))
                      }
                      frame Enabled {
                        n2545 = call-poly <vilib>:"Random Number (Range).vi"("lower bound (0)"=49.89, "upper bound (100)"=50.8) -> ("number"=w3103:dbl)  [unwired: 9 in]
                      }
                    }
                    "StartFlg" <- TRUE ("StartFlg")
                  }
                }
                n2546 = case shown="True" w3057 {
                  frame False {
                  }
                  frame True {
                    n2547 = local write "clk"(10.0 ("clk")) -> ()
                    n2548 = Get Date/Time In Seconds() -> (seconds since 1Jan1904=w3111:timestamp)
                    n2549 = To Double Precision Float(number=w3111) -> (double precision float=w3109:dbl)
                    n2550 = local write "act save time"(w3109) -> ()
                    n2551 = local write "acq timer"(w3109) -> ()
                  }
                }
                n2552 = call "Elapsed Time"("Time Target (s)"="Countdown", "Reset"=w3046) -> ("Elapsed Time (s)"=w3051:dbl, "Time has Elapsed"=w3049:bool)  [unwired: 10 in, 6 out]
                "Countdown 2" <- w3051
                n2553 = Subtract(x=w3051, y=2.0) -> (x-y=w3054:dbl)
                n2554 = Less?(x=w3054, y="Countdown") -> (x < y?=w3052:bool)
                n2555 = And(x=w3052, y=w3049) -> (x .and. y?=w3048:bool)
                n2556 = case shown="True" w3048 {
                  frame False {
                  }
                  frame True {
                    (unwired) dbl[] [] ("History Data")
                    n2557 = local write "Engage"(FALSE ("Engage")) -> ()
                    n2558 = local write "RUN"(TRUE ("RUN")) -> ()
                    n2559 = local read "Humidity ( %RH )"() -> (→"Rh Before":dbl)
                  }
                }
                n2560 = local read "Test \nStatus"() -> (w3044:bool)
                n2561 = Select(t=w3042, s=w3044, f=0.0) -> (s? t:f=w3043:dbl)
                n2562 = local write "Frequency ( Hz )"(w3043) -> ()
              }
              frame #1 {
                w3134 = 1000000.0 ("x")
                # "HC;1/0\nST;VALUE"
                # "Elapsed time\ncof\nstroke\nAir temp\nTemp\nHumidity"
                # "acq timer\n\nact save time"
                # "convert to microseconds"
                n2563 = local read "COUNT"() -> (w3117:i32)
                n2564 = local read "Rate"() -> (w3130:dbl)
                n2565 = Divide(x=w3134, y=w3130) -> (x/y=w3135:dbl)
                n2566 = Greater Or Equal?(x=w3117, y=250) -> (x >= y?=w3116:bool)
                n2567 = Get Date/Time In Seconds() -> (seconds since 1Jan1904=w3137:timestamp)
                n2568 = local read "Samplingtime 2"() -> (w3115:dbl)
                n2569 = local read "act save time"() -> (w3132:dbl)
                n2570 = Divide(x=w3135, y=w3134) -> (x/y=w3133:dbl)
                n2571 = To Double Precision Float(number=w3137) -> (double precision float=w3126:dbl)
                n2572 = Add(x=w3132, y=w3115) -> (x+y=w3131:dbl)
                n2573 = local read "acq timer"() -> (w3136:dbl)
                n2574 = local read "COUNT"() -> (w3119:i32)
                n2575 = Greater Or Equal?(x=w3126, y=w3131) -> (x >= y?=w3114:bool)
                n2576 = Multiply(x=w3133, y=w3119) -> (x*y=w3125:dbl)
                n2577 = Subtract(x=w3126, y=w3136) -> (x-y=w3128:dbl)
                n2578 = case shown="True" w3116 {
                  frame False {
                    n2579 = local read "COUNT"() -> (w3138:i32)
                    n2580 = Increment(x=w3138) -> (x+1=w3139:i32)
                    n2581 = local write "COUNT"(w3139) -> ()
                  }
                  frame True {
                    n2582 = local write "COUNT"(0 ("COUNT")) -> ()
                  }
                }
                n2583 = local read "Save"() -> (w3129:bool)
                n2584 = Add(x=w3128, y=w3125) -> (x+y=w3112:dbl)
                "Elapsed time 3" <- w3112
                n2585 = And(x=w3114, y=w3129) -> (x .and. y?=w3127:bool)
                n2586 = Divide(x=w3112, y=60.0) -> (x/y=w3123:dbl)
                n2587 = local read "Test \nStatus"() -> (w3113:bool)
                n2588 = local read "clk"() -> (w3120:dbl)
                n2589 = Equal?(x=w3120, y=10.0) -> (x = y?=w3122:bool)
                n2590 = case shown="True" w3127 {
                  tunnel: w3126 -> [_ w3259]
                  tunnel: [FALSE ("Boolean 2") TRUE ("Boolean 2")] -> _
                  frame False {
                  }
                  frame True {
                    w3213 = ";" ("Substring")
                    # "Pid out/\nFreq response value"
                    n2591 = local write "act save time"(w3259) -> ()
                    n2592 = local read "FILE"() -> (w3207:string)
                    n2593 = call "file check.vi"("file name in"=w3207) -> ("error out"=w3210:errorcluster, "file name out"=w3205:string)  [unwired: 9 in]
                    n2594 = local read "LVDT STROKE"() -> (w3202:dbl)
                    n2595 = local read "Add up Stroke"() -> (w3200:dbl)
                    n2596 = call "FILE PATH CREATION.vi"("error in"=w3210, "FILE NAME :"=w3205) -> ("FILE OUT"=w3208:path)  [unwired: 8 in, 1 out]
                    n2597 = local read "STROKE Initialize"() -> (w3195:bool)
                    n2598 = Concatenate Strings(w3205, ".dgf" ("Substring")) -> (w3209:string)
                    n2599 = Subtract(x=w3202, y=w3200) -> (x-y=w3201:dbl)
                    n2600 = Absolute Value(x=w3201) -> (abs(x)=w3198:dbl)
                    n2601 = local read "FF 2"() -> (→"Frictional Force ( N )" →"Frictional Force ( N )":dbl)
                    n2602 = Build Path(base path=w3208, name or relative path=w3209) -> (appended path=w3204:path)
                    n2603 = flat-sequence {
                      tunnel: w3198 -> [w3264]
                      tunnel: [w3263] -> w3196
                      tunnel: w3195 -> [w3261]
                      tunnel: [w3266] -> w3197
                      tunnel: w3196 -> [w3266]
                      frame #0 {
                        n2604 = call <vilib>:"Mean PtByPt.vi"("x"=w3264, "sample length"="STROKE FILTER", "initialize"=w3261) -> ("mean"=w3263:dbl)  [unwired: 1 in, 1 out]
                      }
                      frame #1 {
                        "STROKE Initialize" <- FALSE ("STROKE Initialize")
                      }
                    }
                    n2605 = local read "COF 2"() -> (w3218:dbl)
                    "Coefficient of Friction" <- w3218
                    "COF 4" <- w3218
                    "Coefficient of Friction" <- w3218
                    n2606 = local read "TEMP"() -> (w3221:dbl)
                    "Temperature ( Deg C )" <- w3221
                    n2607 = local read "Humidity ( %RH )"() -> (w3220:dbl)
                    "Humidity ( %RH ) 2" <- w3220
                    n2608 = local read "Frequency ( Hz )"() -> (w3227:dbl)
                    n2609 = local read "LVDT STROKE DISPLAY"() -> (w3199:dbl)
                    n2610 = local read "Elapsed time"() -> (w3252:dbl)
                    n2611 = local read "AIR TEMP"() -> (w3225:dbl)
                    n2612 = local read "PID-out"() -> (w3230:dbl)
                    n2613 = local write "Temperature ( Deg C )"(w3221) -> ()
                    n2614 = Number To Fractional String(number=w3199, width (-)=i16 9 ("precision (6)"), precision (6)=i16 6) -> (F-format string=w3245:string)  [unwired: 1 in]
                    n2615 = Number To Fractional String(number=w3225, width (-)=i16 9 ("precision (6)"), precision (6)=i16 3) -> (F-format string=w3244:string)  [unwired: 1 in]
                    n2616 = Number To Fractional String(number=w3221, width (-)=i16 9 ("precision (6)"), precision (6)=i16 3) -> (F-format string=w3241:string)  [unwired: 1 in]
                    n2617 = Number To Fractional String(number=w3220, width (-)=i16 9 ("precision (6)"), precision (6)=i16 3) -> (F-format string=w3238:string)  [unwired: 1 in]
                    n2618 = Number To Fractional String(number=0.0, width (-)=i16 9 ("precision (6)"), precision (6)=i16 3) -> (F-format string=w3235:string)  [unwired: 1 in]
                    n2619 = Number To Fractional String(number=w3230, width (-)=i16 9 ("precision (6)"), precision (6)=i16 3) -> (F-format string=w3231:string)  [unwired: 1 in]
                    n2620 = Number To Fractional String(number=w3227, width (-)=i16 9 ("precision (6)"), precision (6)=i16 3) -> (F-format string=w3226:string)  [unwired: 1 in]
                    n2621 = Number To Fractional String(number=w3218, width (-)=i16 9 ("precision (6)"), precision (6)=i16 6) -> (F-format string=w3253:string)  [unwired: 1 in]
                    n2622 = Number To Fractional String(number=w3252, width (-)=i16 14 ("precision (6)"), precision (6)=i16 3) -> (F-format string=w3254:string)  [unwired: 1 in]
                    n2623 = Bundle("y"=1.02, "LVDT STROKE DISPLAY"=w3199, "y"=0.98) -> (w3219:T31)  [unwired: 1 in]
                    n2624 = Number To Fractional String(number="Ambient Humidity :", width (-)=i16 9 ("precision (6)"), precision (6)=i16 6) -> (F-format string=w3211:string)  [unwired: 1 in]
                    n2625 = local read "RUN"() -> (w3217:bool)
                    n2626 = case shown="True" w3217 {
                      tunnel: w3219 -> [_ w3270]
                      tunnel: w3199 -> [_ w3269]
                      tunnel: w3199 -> [_ w3267]
                      tunnel: w3199 -> [_ w3268]
                      frame False {
                      }
                      frame True {
                        "Stroke ( mm )" <- w3270
                        "Stroke ( mm )" <- w3270
                        "Stroke 4" <- w3269
                        "Stroke 3" <- w3267
                        "Stroke 2" <- w3268
                        "measured_stroke" <- w3267
                      }
                    }
                    n2627 = Concatenate Strings(w3254, w3213, w3253, w3213, w3245, w3213, w3244, w3213, w3241, w3213, w3238, w3213, w3235, w3213, w3231, w3213, w3226, w3213, w3211, "\r") -> (w3251:string)
                    n2628 = call <vilib>:"Write Characters To File.vi"("append to file? (new file:F)"=TRUE, "character string"=w3251, "file path (dialog if empty)"=w3204) -> ()  [unwired: 2 in, 1 out]
                    "refresh flag" <- TRUE ("refresh flag")
                    "LVDT STROKE Actual" <- w3197
                  }
                }
                n2629 = case shown="True" w3113 {
                  tunnel: w3123 -> [_ w3149]
                  tunnel: w3128 -> [_ w3159]
                  tunnel: [0.0 w3155] -> _
                  tunnel: w3122 -> [_ w3154]
                  tunnel: [0.0 w3153] -> _
                  tunnel: w3112 -> [_ w3153]
                  tunnel: w3126 -> [w3142 _]